vi "Dresden R2R Sputter 03.02.2018 IY24.vi"() -> ()   [LabVIEW 2009] (continued)
                      frame #2 {
                        n23216 = local read "Semi"() -> (w28558:bool)
                        n23217 = case shown="False" w28558 {
                          frame #0 {
                            n23218 = local write "RC_5"(TRUE ("RC_2")) -> ()
                            n23219 = Wait (ms)(milliseconds to wait=u32 200 ("millisecond multiple")) -> ()  [unwired: 1 out]
                          }
                          frame #1 {
                          }
                        }
                      }
                    }
                  }
                  frame #1 {
                  }
                }
              }
              frame #6 {
                # "PET COOL UP-CH2"
                n23220 = local read "Semi"() -> (w28561:bool)
                n23221 = case shown="False" w28561 {
                  frame #0 {
                    n23222 = stacked-sequence {
                      frame #0 {
                        n23223 = local read "Semi"() -> (w28562:bool)
                        n23224 = case shown="False" w28562 {
                          frame #0 {
                            n23225 = local write "Ch2_Pet_cool_down_do"(FALSE ("Ch1_pet_cool_up_do")) -> ()
                          }
                          frame #1 {
                          }
                        }
                      }
                      frame #1 {
                        n23226 = local read "Semi"() -> (w28564:bool)
                        n23227 = case shown="False" w28564 {
                          frame #0 {
                            n23228 = while {
                              i -> [w28570]
                              stop <- w28565 stop-if-true
                              n23229 = Greater?(x=w28570, y=200) -> (0:w28569:bool)
                              n23230 = case shown="True" w28569 {
                                frame #0 {
                                }
                                frame #1 {
                                n23231 = local write "Error Message"("" ("Error Message")) -> ()
                                n23232 = local write "Semi"(TRUE ("Semi")) -> ()
                                }
                              }
                              n23233 = local read "Ch2_Pet_cool_up_di"() -> (w28568:bool)
                              n23234 = case shown="False" w28568 {
                                tunnel: [FALSE TRUE] -> w28567
                                frame #0 {
                                n23235 = Wait Until Next ms Multiple(millisecond multiple=u32 200) -> ()  [unwired: 1 out]
                                n23236 = local write "Ch2_Pet_cool_up_do"(TRUE ("Ch1_pet_cool_up_do")) -> ()
                                }
                                frame #1 {
                                }
                              }
                              n23237 = local read "Semi"() -> (w28566:bool)
                              n23238 = Or(x=w28567, y=w28566) -> (x .or. y?=w28565:bool)
                            }
                          }
                          frame #1 {
                          }
                        }
                      }
                      frame #2 {
                        n23239 = local read "Semi"() -> (w28578:bool)
                        n23240 = case shown="False" w28578 {
                          frame #0 {
                            n23241 = local write "RC_6"(TRUE ("RC_2")) -> ()
                            n23242 = Wait (ms)(milliseconds to wait=u32 200 ("millisecond multiple")) -> ()  [unwired: 1 out]
                          }
                          frame #1 {
                          }
                        }
                      }
                    }
                  }
                  frame #1 {
                  }
                }
              }
              frame #7 {
                # "PET COOL UP-CH3"
                n23243 = local read "Semi"() -> (w28581:bool)
                n23244 = case shown="False" w28581 {
                  frame #0 {
                    n23245 = stacked-sequence {
                      frame #0 {
                        n23246 = local read "Semi"() -> (w28582:bool)
                        n23247 = case shown="False" w28582 {
                          frame #0 {
                            n23248 = local write "Ch3_Pet_cool_down_do"(FALSE ("Ch1_pet_cool_up_do")) -> ()
                          }
                          frame #1 {
                          }
                        }
                      }
                      frame #1 {
                        n23249 = local read "Semi"() -> (w28584:bool)
                        n23250 = case shown="False" w28584 {
                          frame #0 {
                            n23251 = while {
                              i -> [w28590]
                              stop <- w28585 stop-if-true
                              n23252 = Greater?(x=w28590, y=200) -> (0:w28589:bool)
                              n23253 = case shown="True" w28589 {
                                frame #0 {
                                }
                                frame #1 {
                                n23254 = local write "Error Message"("" ("Error Message")) -> ()
                                n23255 = local write "Semi"(TRUE ("Semi")) -> ()
                                }
                              }
                              n23256 = local read "Ch3_Pet_cool_up_di"() -> (w28588:bool)
                              n23257 = case shown="False" w28588 {
                                tunnel: [FALSE TRUE] -> w28587
                                frame #0 {
                                n23258 = Wait Until Next ms Multiple(millisecond multiple=u32 200) -> ()  [unwired: 1 out]
                                n23259 = local write "Ch3_Pet_cool_up_do"(TRUE ("Ch1_pet_cool_up_do")) -> ()
                                }
                                frame #1 {
                                }
                              }
                              n23260 = local read "Semi"() -> (w28586:bool)
                              n23261 = Or(x=w28587, y=w28586) -> (x .or. y?=w28585:bool)
                            }
                          }
                          frame #1 {
                          }
                        }
                      }
                      frame #2 {
                        n23262 = local read "Semi"() -> (w28598:bool)
                        n23263 = case shown="False" w28598 {
                          frame #0 {
                            n23264 = local write "RC_7"(TRUE ("RC_2")) -> ()
                            n23265 = Wait (ms)(milliseconds to wait=u32 200 ("millisecond multiple")) -> ()  [unwired: 1 out]
                          }
                          frame #1 {
                          }
                        }
                      }
                    }
                  }
                  frame #1 {
                  }
                }
              }
              frame #8 {
                # "PET COOL UP-CH4"
                n23266 = local read "Semi"() -> (w28601:bool)
                n23267 = case shown="False" w28601 {
                  frame #0 {
                    n23268 = stacked-sequence {
                      frame #0 {
                        n23269 = local read "Semi"() -> (w28602:bool)
                        n23270 = case shown="False" w28602 {
                          frame #0 {
                            n23271 = local write "Ch4_Pet_cool_down_do"(FALSE ("Ch1_pet_cool_up_do")) -> ()
                          }
                          frame #1 {
                          }
                        }
                      }
                      frame #1 {
                        n23272 = local read "Semi"() -> (w28604:bool)
                        n23273 = case shown="False" w28604 {
                          frame #0 {
                            n23274 = while {
                              i -> [w28610]
                              stop <- w28605 stop-if-true
                              n23275 = Greater?(x=w28610, y=200) -> (0:w28609:bool)
                              n23276 = case shown="True" w28609 {
                                frame #0 {
                                }
                                frame #1 {
                                n23277 = local write "Error Message"("" ("Error Message")) -> ()
                                n23278 = local write "Semi"(TRUE ("Semi")) -> ()
                                }
                              }
                              n23279 = local read "Ch4_Pet_cool_up_di"() -> (w28608:bool)
                              n23280 = case shown="False" w28608 {
                                tunnel: [FALSE TRUE] -> w28607
                                frame #0 {
                                n23281 = Wait Until Next ms Multiple(millisecond multiple=u32 200) -> ()  [unwired: 1 out]
                                n23282 = local write "Ch4_Pet_cool_up_do"(TRUE ("Ch1_pet_cool_up_do")) -> ()
                                }
                                frame #1 {
                                }
                              }
                              n23283 = local read "Semi"() -> (w28606:bool)
                              n23284 = Or(x=w28607, y=w28606) -> (x .or. y?=w28605:bool)
                            }
                          }
                          frame #1 {
                          }
                        }
                      }
                      frame #2 {
                        n23285 = local read "Semi"() -> (w28618:bool)
                        n23286 = case shown="False" w28618 {
                          frame #0 {
                            n23287 = local write "RC_8"(TRUE ("RC_2")) -> ()
                            n23288 = Wait (ms)(milliseconds to wait=u32 200 ("millisecond multiple")) -> ()  [unwired: 1 out]
                          }
                          frame #1 {
                          }
                        }
                      }
                    }
                  }
                  frame #1 {
                  }
                }
              }
              frame #9 {
                # "CST FIX-UP CH1"
                n23289 = local read "Semi"() -> (w28621:bool)
                n23290 = case shown="False" w28621 {
                  frame #0 {
                    n23291 = stacked-sequence {
                      frame #0 {
                        n23292 = local read "Semi"() -> (w28622:bool)
                        n23293 = case shown="False" w28622 {
                          frame #0 {
                            n23294 = while {
                              i -> [w28628]
                              stop <- w28623 stop-if-true
                              n23295 = Greater?(x=w28628, y=100) -> (0:w28627:bool)
                              n23296 = case shown="True" w28627 {
                                frame #0 {
                                }
                                frame #1 {
                                n23297 = local write "Error Message"("" ("Error Message")) -> ()
                                n23298 = local write "Semi"(TRUE ("Semi")) -> ()
                                }
                              }
                              n23299 = local read "Ch1_Cst_fix_up_di"() -> (w28626:bool)
                              n23300 = case shown="True" w28626 {
                                tunnel: [FALSE TRUE] -> w28625
                                frame #0 {
                                n23301 = Wait Until Next ms Multiple(millisecond multiple=u32 200) -> ()  [unwired: 1 out]
                                n23302 = local write "Ch1_Cst_fix_do"(FALSE ("Ch1_pet_cool_up_do")) -> ()
                                }
                                frame #1 {
                                }
                              }
                              n23303 = local read "Semi"() -> (w28624:bool)
                              n23304 = Or(x=w28625, y=w28624) -> (x .or. y?=w28623:bool)
                            }
                          }
                          frame #1 {
                          }
                        }
                      }
                      frame #1 {
                        n23305 = local read "Semi"() -> (w28636:bool)
                        n23306 = case shown="False" w28636 {
                          frame #0 {
                            n23307 = Wait (ms)(milliseconds to wait=u32 200 ("millisecond multiple")) -> ()  [unwired: 1 out]
                            n23308 = local write "RC_9"(TRUE ("RC_2")) -> ()
                          }
                          frame #1 {
                          }
                        }
                      }
                    }
                  }
                  frame #1 {
                  }
                }
              }
              frame #10 {
                # "CST FIX-UP CH2"
                n23309 = local read "Semi"() -> (w28639:bool)
                n23310 = case shown="False" w28639 {
                  frame #0 {
                    n23311 = stacked-sequence {
                      frame #0 {
                        n23312 = local read "Semi"() -> (w28640:bool)
                        n23313 = case shown="False" w28640 {
                          frame #0 {
                            n23314 = while {
                              i -> [w28646]
                              stop <- w28641 stop-if-true
                              n23315 = Greater?(x=w28646, y=100) -> (0:w28645:bool)
                              n23316 = case shown="True" w28645 {
                                frame #0 {
                                }
                                frame #1 {
                                n23317 = local write "Error Message"("" ("Error Message")) -> ()
                                n23318 = local write "Semi"(TRUE ("Semi")) -> ()
                                }
                              }
                              n23319 = local read "Ch2_Cst_fix_up_di"() -> (w28644:bool)
                              n23320 = case shown="False" w28644 {
                                tunnel: [FALSE TRUE] -> w28643
                                frame #0 {
                                n23321 = Wait Until Next ms Multiple(millisecond multiple=u32 200) -> ()  [unwired: 1 out]
                                n23322 = local write "Ch2_Cst_fix_do"(FALSE ("Ch1_pet_cool_up_do")) -> ()
                                }
                                frame #1 {
                                }
                              }
                              n23323 = local read "Semi"() -> (w28642:bool)
                              n23324 = Or(x=w28643, y=w28642) -> (x .or. y?=w28641:bool)
                            }
                          }
                          frame #1 {
                          }
                        }
                      }
                      frame #1 {
                        n23325 = local read "Semi"() -> (w28654:bool)
                        n23326 = case shown="False" w28654 {
                          frame #0 {
                            n23327 = local write "RC_10"(TRUE ("RC_2")) -> ()
                            n23328 = Wait (ms)(milliseconds to wait=u32 200 ("millisecond multiple")) -> ()  [unwired: 1 out]
                          }
                          frame #1 {
                          }
                        }
                      }
                    }
                  }
                  frame #1 {
                  }
                }
              }
              frame #11 {
                # "CST FIX-UP CH3"
                n23329 = local read "Semi"() -> (w28657:bool)
                n23330 = case shown="False" w28657 {
                  frame #0 {
                    n23331 = stacked-sequence {
                      frame #0 {
                        n23332 = local read "Semi"() -> (w28658:bool)
                        n23333 = case shown="False" w28658 {
                          frame #0 {
                            n23334 = while {
                              i -> [w28664]
                              stop <- w28659 stop-if-true
                              n23335 = Greater?(x=w28664, y=100) -> (0:w28663:bool)
                              n23336 = case shown="True" w28663 {
                                frame #0 {
                                }
                                frame #1 {
                                n23337 = local write "Error Message"("" ("Error Message")) -> ()
                                n23338 = local write "Semi"(TRUE ("Semi")) -> ()
                                }
                              }
                              n23339 = local read "Ch3_Cst_fix_up_di"() -> (w28662:bool)
                              n23340 = case shown="False" w28662 {
                                tunnel: [FALSE TRUE] -> w28661
                                frame #0 {
                                n23341 = Wait Until Next ms Multiple(millisecond multiple=u32 200) -> ()  [unwired: 1 out]
                                n23342 = local write "Ch3_Cst_fix_do"(FALSE ("Ch1_pet_cool_up_do")) -> ()
                                }
                                frame #1 {
                                }
                              }
                              n23343 = local read "Semi"() -> (w28660:bool)
                              n23344 = Or(x=w28661, y=w28660) -> (x .or. y?=w28659:bool)
                            }
                          }
                          frame #1 {
                          }
                        }
                      }
                      frame #1 {
                        n23345 = local read "Semi"() -> (w28672:bool)
                        n23346 = case shown="False" w28672 {
                          frame #0 {
                            n23347 = local write "RC_11"(TRUE ("RC_2")) -> ()
                            n23348 = Wait (ms)(milliseconds to wait=u32 200 ("millisecond multiple")) -> ()  [unwired: 1 out]
                          }
                          frame #1 {
                          }
                        }
                      }
                    }
                  }
                  frame #1 {
                  }
                }
              }
              frame #12 {
                # "CST FIX-UP CH4"
                n23349 = local read "Semi"() -> (w28675:bool)
                n23350 = case shown="False" w28675 {
                  frame #0 {
                    n23351 = stacked-sequence {
                      frame #0 {
                        n23352 = local read "Semi"() -> (w28676:bool)
                        n23353 = case shown="False" w28676 {
                          frame #0 {
                            n23354 = while {
                              i -> [w28682]
                              stop <- w28677 stop-if-true
                              n23355 = Greater?(x=w28682, y=100) -> (0:w28681:bool)
                              n23356 = case shown="True" w28681 {
                                frame #0 {
                                }
                                frame #1 {
                                n23357 = local write "Error Message"("" ("Error Message")) -> ()
                                n23358 = local write "Semi"(TRUE ("Semi")) -> ()
                                }
                              }
                              n23359 = local read "Ch4_Cst_fix_up_di"() -> (w28680:bool)
                              n23360 = case shown="False" w28680 {
                                tunnel: [FALSE TRUE] -> w28679
                                frame #0 {
                                n23361 = Wait Until Next ms Multiple(millisecond multiple=u32 200) -> ()  [unwired: 1 out]
                                n23362 = local write "Ch4_Cst_fix_do"(FALSE ("Ch1_pet_cool_up_do")) -> ()
                                }
                                frame #1 {
                                }
                              }
                              n23363 = local read "Semi"() -> (w28678:bool)
                              n23364 = Or(x=w28679, y=w28678) -> (x .or. y?=w28677:bool)
                            }
                          }
                          frame #1 {
                          }
                        }
                      }
                      frame #1 {
                        n23365 = local read "Semi"() -> (w28690:bool)
                        n23366 = case shown="False" w28690 {
                          frame #0 {
                            n23367 = Wait (ms)(milliseconds to wait=u32 200 ("millisecond multiple")) -> ()  [unwired: 1 out]
                            n23368 = local write "RC_12"(TRUE ("RC_2")) -> ()
                          }
                          frame #1 {
                          }
                        }
                      }
                      frame #2 {
                        n23369 = local read "Semi"() -> (w28693:bool)
                        n23370 = case shown="False" w28693 {
                          frame #0 {
                            n23371 = local write "Routine_check_transfer"(FALSE ("Routine_check_transfer")) -> ()
                            n23372 = Wait (ms)(milliseconds to wait=u32 200 ("millisecond multiple")) -> ()  [unwired: 1 out]
                          }
                          frame #1 {
                          }
                        }
                      }
                    }
                  }
                  frame #1 {
                  }
                }
              }
            }
          }
          frame #1 {
          }
        }
      }
    }
  }
  n23373 = while {
    stop <- FALSE stop-if-true
    n23374 = Wait Until Next ms Multiple(millisecond multiple=u32 300) -> ()  [unwired: 1 out]
    n23375 = case shown="True" "Couple" {
      frame #0 {
      }
      frame #1 {
        n23376 = stacked-sequence {
          frame #0 {
            n23377 = local read "Semi"() -> (w28744:bool)
            n23378 = case shown="False" w28744 {
              frame #0 {
                n23379 = while {
                  i -> [w28751]
                  stop <- w28746 stop-if-true
                  n23380 = Greater?(x=w28751, y=50) -> (0:w28749:bool)
                  n23381 = local read "Ch1_Cst_fix_down_di"() -> (w28745:bool)
                  n23382 = case shown="True" w28749 {
                    frame #0 {
                    }
                    frame #1 {
                      n23383 = local write "Semi"(TRUE ("Semi")) -> ()
                      n23384 = local write "Error Message"("Up/Down positions could not reach\nthe down position.\nPlease check connections." ("Error Message")) -> ()
                    }
                  }
                  n23385 = case shown="False" w28745 {
                    tunnel: [FALSE TRUE] -> w28748
                    frame #0 {
                      n23386 = Wait Until Next ms Multiple(millisecond multiple=u32 200) -> ()  [unwired: 1 out]
                      n23387 = local write "Ch1_Cst_fix_do"(TRUE ("Ch1_pet_cool_up_do")) -> ()
                    }
                    frame #1 {
                    }
                  }
                  n23388 = local read "Semi"() -> (w28747:bool)
                  n23389 = Or(x=w28748, y=w28747) -> (x .or. y?=w28746:bool)
                }
              }
              frame #1 {
              }
            }
          }
          frame #1 {
            n23390 = local read "Semi"() -> (w28758:bool)
            n23391 = case shown="False" w28758 {
              frame #0 {
                n23392 = local write "Ch1_Pet_cool_up_do"(FALSE ("Ch1_pet_cool_up_do")) -> ()
              }
              frame #1 {
              }
            }
          }
          frame #2 {
            n23393 = while {
              i -> [w28766]
              stop <- w28761 stop-if-true
              n23394 = Greater?(x=w28766, y=300) -> (0:w28764:bool)
              n23395 = case shown="True" w28764 {
                frame #0 {
                }
                frame #1 {
                  n23396 = local write "Semi"(TRUE ("Semi")) -> ()
                  n23397 = local write "Error Message"("SBS Cool Up/Down positions could not reach\nthe down position.\nPlease check connections." ("Error Message")) -> ()
                }
              }
              n23398 = local read "Ch1_Pet_cool_down_di"() -> (w28760:bool)
              n23399 = case shown="False" w28760 {
                tunnel: [FALSE TRUE] -> w28763
                frame #0 {
                  n23400 = Wait Until Next ms Multiple(millisecond multiple=u32 200) -> ()  [unwired: 1 out]
                  n23401 = local write "Ch1_Pet_cool_down_do"(TRUE ("Ch1_pet_cool_up_do")) -> ()
                }
                frame #1 {
                }
              }
              n23402 = local read "Semi"() -> (w28762:bool)
              n23403 = Or(x=w28763, y=w28762) -> (x .or. y?=w28761:bool)
            }
          }
          frame #3 {
            n23404 = local read "Semi"() -> (w28773:bool)
            n23405 = case shown="False" w28773 {
              frame #0 {
                n23406 = local write "Ch1_SRV1_PIST_Back_do"(FALSE ("Ch1_pet_cool_up_do")) -> ()
              }
              frame #1 {
              }
            }
          }
          frame #4 {
            n23407 = while {
              i -> [w28780]
              stop <- w28775 stop-if-true
              n23408 = Greater?(x=w28780, y=100) -> (0:w28779:bool)
              n23409 = case shown="True" w28779 {
                frame #0 {
                }
                frame #1 {
                  n23410 = local write "Error Message"("" ("Error Message")) -> ()
                  n23411 = local write "Semi"(TRUE ("Semi")) -> ()
                }
              }
              n23412 = local read "Ch1_SRV1_PIST For_di"() -> (w28778:bool)
              n23413 = case shown="False" w28778 {
                tunnel: [FALSE TRUE] -> w28777
                frame #0 {
                  n23414 = local write "Ch1_SRV1_PIST For_do"(TRUE ("Ch1_pet_cool_up_do")) -> ()
                  n23415 = Wait Until Next ms Multiple(millisecond multiple=u32 200) -> ()  [unwired: 1 out]
                }
                frame #1 {
                }
              }
              n23416 = local read "Semi"() -> (w28776:bool)
              n23417 = Or(x=w28777, y=w28776) -> (x .or. y?=w28775:bool)
            }
          }
        }
      }
    }
    n23418 = case shown="True" "Decouple" {
      frame #0 {
      }
      frame #1 {
        n23419 = stacked-sequence {
          frame #0 {
            n23420 = local read "Semi"() -> (w28700:bool)
            n23421 = case shown="False" w28700 {
              frame #0 {
                n23422 = while {
                  i -> [w28707]
                  stop <- w28702 stop-if-true
                  n23423 = Greater?(x=w28707, y=50) -> (0:w28705:bool)
                  n23424 = local read "Ch1_Cst_fix_up_di"() -> (w28701:bool)
                  n23425 = case shown="True" w28705 {
                    frame #0 {
                    }
                    frame #1 {
                      n23426 = local write "Semi"(TRUE ("Semi")) -> ()
                      n23427 = local write "Error Message"("Up/Down positions could not reach\nthe down position.\nPlease check connections." ("Error Message")) -> ()
                    }
                  }
                  n23428 = case shown="False" w28701 {
                    tunnel: [FALSE TRUE] -> w28704
                    frame #0 {
                      n23429 = Wait Until Next ms Multiple(millisecond multiple=u32 200) -> ()  [unwired: 1 out]
                      n23430 = local write "Ch1_Cst_fix_do"(FALSE ("Ch1_pet_cool_up_do")) -> ()
                    }
                    frame #1 {
                    }
                  }
                  n23431 = local read "Semi"() -> (w28703:bool)
                  n23432 = Or(x=w28704, y=w28703) -> (x .or. y?=w28702:bool)
                }
              }
              frame #1 {
              }
            }
          }
          frame #1 {
            n23433 = local read "Semi"() -> (w28714:bool)
            n23434 = case shown="False" w28714 {
              frame #0 {
                n23435 = local write "Ch1_Pet_cool_down_do"(FALSE ("Ch1_pet_cool_up_do")) -> ()
              }
              frame #1 {
              }
            }
          }
          frame #2 {
            n23436 = while {
              i -> [w28722]
              stop <- w28717 stop-if-true
              n23437 = Greater?(x=w28722, y=300) -> (0:w28720:bool)
              n23438 = case shown="True" w28720 {
                frame #0 {
                }
                frame #1 {
                  n23439 = local write "Semi"(TRUE ("Semi")) -> ()
                  n23440 = local write "Error Message"("SBS Cool Up/Down positions could not reach\nthe down position.\nPlease check connections." ("Error Message")) -> ()
                }
              }
              n23441 = local read "Ch1_Pet_cool_up_di"() -> (w28716:bool)
              n23442 = case shown="False" w28716 {
                tunnel: [FALSE TRUE] -> w28719
                frame #0 {
                  n23443 = Wait Until Next ms Multiple(millisecond multiple=u32 200) -> ()  [unwired: 1 out]
                  n23444 = local write "Ch1_Pet_cool_up_do"(TRUE ("Ch1_pet_cool_up_do")) -> ()
                }
                frame #1 {
                }
              }
              n23445 = local read "Semi"() -> (w28718:bool)
              n23446 = Or(x=w28719, y=w28718) -> (x .or. y?=w28717:bool)
            }
          }
          frame #3 {
            n23447 = local read "Semi"() -> (w28729:bool)
            n23448 = case shown="False" w28729 {
              frame #0 {
                n23449 = local write "Ch1_SRV1_PIST For_do"(FALSE ("Ch1_pet_cool_up_do")) -> ()
              }
              frame #1 {
              }
            }
          }
          frame #4 {
            n23450 = while {
              i -> [w28736]
              stop <- w28731 stop-if-true
              n23451 = Greater?(x=w28736, y=100) -> (0:w28735:bool)
              n23452 = case shown="True" w28735 {
                frame #0 {
                }
                frame #1 {
                  n23453 = local write "Error Message"("" ("Error Message")) -> ()
                  n23454 = local write "Semi"(TRUE ("Semi")) -> ()
                }
              }
              n23455 = local read "Ch1_SRV1_PIST_Back_di"() -> (w28734:bool)
              n23456 = case shown="False" w28734 {
                tunnel: [FALSE TRUE] -> w28733
                frame #0 {
                  n23457 = local write "Ch1_SRV1_PIST_Back_do"(TRUE ("Ch1_pet_cool_up_do")) -> ()
                  n23458 = Wait Until Next ms Multiple(millisecond multiple=u32 200) -> ()  [unwired: 1 out]
                }
                frame #1 {
                }
              }
              n23459 = local read "Semi"() -> (w28732:bool)
              n23460 = Or(x=w28733, y=w28732) -> (x .or. y?=w28731:bool)
            }
          }
        }
      }
    }
  }
  n23461 = VISA Close(VISA resource name=w789, error in (no error)=w788) -> ()  [unwired: 1 out]
  n23462 = while {
    stop <- i16? 0 stop-if-true
    n23463 = Wait (ms)(milliseconds to wait=i32? 300) -> ()  [unwired: 1 out]
    n23464 = stacked-sequence {
      frame #0 {
        n23465 = case shown="True" "Clean_Pumping_ch1" {
          frame #0 {
          }
          frame #1 {
            w28830 = i16? 0
            n23466 = local write "Clean_Pumping_ch1"(w28830) -> ()
            "Ch1_PV2" <- w28830
            "Ch1_PV6" <- w28830
            "Ch1_PV7" <- w28830
            "Ch1_PV8" <- w28830
            "Ch1_PV9" <- w28830
            "Ch1_PV15" <- w28830
            "Ch1_PV10" <- w28830
            "Ch1_PV16" <- w28830
            "Ch1_PV13" <- w28830
            "Ch1_PA15" <- w28830
            "Ch1_PA9" <- w28830
            "Ch1_PA10" <- w28830
            "Ch1_PA17" <- w28830
            "Ch1_PA2" <- w28830
            "Ch1_PA6" <- w28830
            "Ch1_PA7" <- w28830
            "Ch1_PA8" <- w28830
            "Ch1_PA14" <- w28830
            "Ch1_PA19" <- w28830
            "Ch1_PA20" <- w28830
            "Ch1_PA24" <- w28830
            "Ch1_PA25" <- w28830
            "Ch1_PA16" <- w28830
            "Ch1_PA18" <- w28830
            "Ch1_PA22" <- w28830
            "Ch1_PV11" <- w28830
            "Ch1_PV14" <- w28830
            "Ch1_PV19" <- w28830
            "Ch1_PV20" <- w28830
            "Ch1_PV23" <- w28830
            "Ch1_PV22" <- w28830
            "Ch1_PV4" <- w28830
            "Ch1_PV18" <- w28830
            "Ch1_PA4" <- w28830
            "Ch1_PA11" <- w28830
            "Ch1_PA13" <- w28830
            "Ch1_PA21" <- w28830
            "Ch1_PV12" <- w28830
            "Ch1_PV17" <- w28830
            "Ch1_PA26" <- w28830
            "Ch1_PA27" <- w28830
            "Ch1_PA28" <- w28830
            "Ch1_PA30" <- w28830
            "Ch1_PA29" <- w28830
            "Ch1_PA12" <- w28830
            "Ch1_PA23" <- w28830
            "Ch1_PA31" <- w28830
            "Ch1_PV3" <- w28830
            "Ch1_PA3" <- w28830
            "Ch1_PV1" <- w28830
            "Ch1_PA1" <- w28830
            "Ch1_PA5" <- w28830
            "Ch1_PV5" <- w28830
            "Ch1_PA33" <- w28830
            "Ch1_PA34" <- w28830
            "Ch1_PA32" <- w28830
            "Ch1_PV21" <- w28830
          }
        }
        n23467 = case shown="True" "Clean_shutdown_ch1" {
          frame #0 {
          }
          frame #1 {
            w28831 = i16? 0
            n23468 = local write "Clean_shutdown_ch1"(w28831) -> ()
            "Ch1_Sd0" <- w28831
            "Ch1_Sd1" <- w28831
            "Ch1_Sd3" <- w28831
            "Ch1_Sd8" <- w28831
            "Ch1_Sd6" <- w28831
            "Ch1_Sd5" <- w28831
            "Ch1_Sd14" <- w28831
            "Ch1_Sd7" <- w28831
            "Ch1_Sd10" <- w28831
            "Ch1_Sd12" <- w28831
            "Ch1_Sd11" <- w28831
            "Ch1_Sd19" <- w28831
            "Ch1_Sd4" <- w28831
            "Ch1_Sd17" <- w28831
            "Ch1_Sd2" <- w28831
            "Ch1_Sd16" <- w28831
            "Ch1_Sd18" <- w28831
            "Ch1_Sd13" <- w28831
            "Ch1_Sd15" <- w28831
            "Ch1_Sd9" <- w28831
          }
        }
      }
    }
    n23469 = stacked-sequence {
      frame #0 {
        n23470 = case shown="True" "Clean_Pumping_ch2" {
          frame #0 {
          }
          frame #1 {
            w28827 = i16? 0
            n23471 = local write "Clean_Pumping_ch2"(w28827) -> ()
            "Ch2_PA0" <- w28827
            "Ch2_PA1" <- w28827
            "Ch2_PA2" <- w28827
            "Ch2_PA3" <- w28827
            "Ch2_PA4" <- w28827
            "Ch2_PA5" <- w28827
            "Ch2_PA6" <- w28827
            "Ch2_PA7" <- w28827
            "Ch2_PA8" <- w28827
            "Ch2_PA9" <- w28827
            "Ch2_PA10" <- w28827
            "Ch2_PA11" <- w28827
            "Ch2_PA12" <- w28827
            "Ch2_PA13" <- w28827
            "Ch2_PA18" <- w28827
            "Ch2_PA14" <- w28827
            "Ch2_PA15" <- w28827
            "Ch2_PA17" <- w28827
            "Ch2_PA16" <- w28827
            "Ch2_PA19" <- w28827
            "Ch2_PA20" <- w28827
            "Ch2_PA21" <- w28827
            "Ch2_PA22" <- w28827
            "Ch2_PA23" <- w28827
            "Ch2_PA24" <- w28827
            "Ch2_PA25" <- w28827
            "Ch2_PA26" <- w28827
            "Ch2_PA27" <- w28827
            "Ch2_PA28" <- w28827
            "Ch2_PA29" <- w28827
            "Ch2_PA30" <- w28827
            "Ch2_PA31" <- w28827
            "Ch2_PA32" <- w28827
            "Ch2_PA35" <- w28827
            "Ch2_PV0" <- w28827
            "Ch2_PV1" <- w28827
            "Ch2_PV7" <- w28827
            "Ch2_PV2" <- w28827
            "Ch2_PV3" <- w28827
            "Ch2_PV4" <- w28827
            "Ch2_PV5" <- w28827
            "Ch2_PV6" <- w28827
            "Ch2_PV8" <- w28827
            "Ch2_PV9" <- w28827
            "Ch2_PV10" <- w28827
            "Ch2_PV11" <- w28827
            "Ch2_PV12" <- w28827
            "Ch2_PV13" <- w28827
            "Ch2_PV14" <- w28827
            "Ch2_PV15" <- w28827
            "Ch2_PV16" <- w28827
            "Ch2_PV17" <- w28827
            "Ch2_PV18" <- w28827
            "Ch2_PV19" <- w28827
            "Ch2_PV20" <- w28827
            "Ch2_PV24" <- w28827
            "Ch2_PV21" <- w28827
            "Ch2_PV25" <- w28827
            "Ch2_PA36" <- w28827
            "Ch2_PA33" <- w28827
            "Ch2_PA34" <- w28827
            "Ch2_PV22" <- w28827
            "Ch2_PV23" <- w28827
          }
        }
        n23472 = case shown="True" "Clean_shutdown_ch2" {
          frame #0 {
          }
          frame #1 {
            w28826 = i16? 0
            n23473 = local write "Clean_shutdown_ch2"(w28826) -> ()
            "Ch2_Sd1" <- w28826
            "Ch2_Sd3" <- w28826
            "Ch2_Sd2" <- w28826
            "Ch2_Sd4" <- w28826
            "Ch2_Sd5" <- w28826
            "Ch2_Sd7" <- w28826
            "Ch2_Sd6" <- w28826
            "Ch2_Sd8" <- w28826
            "Ch2_Sd9" <- w28826
            "Ch2_Sd10" <- w28826
            "Ch2_Sd11" <- w28826
            "Ch2_Sd12" <- w28826
            "Ch2_Sd13" <- w28826
            "Ch2_Sd14" <- w28826
            "Ch2_Sd17" <- w28826
            "Ch2_Sd18" <- w28826
            "Ch2_Sd19" <- w28826
            "Ch2_Sd20" <- w28826
            "Ch2_Sd21" <- w28826
            "Ch2_Sd22" <- w28826
            "Ch2_Sd15" <- w28826
            "Ch2_Sd16" <- w28826
          }
        }
      }
    }
    n23474 = stacked-sequence {
      frame #0 {
        n23475 = case shown="True" "Clean_Pumping_ch3" {
          frame #0 {
          }
          frame #1 {
            w28823 = i16? 0
            n23476 = local write "Clean_Pumping_ch3"(w28823) -> ()
            "Ch3_PA0" <- w28823
            "Ch3_PA1" <- w28823
            "Ch3_PA2" <- w28823
            "Ch3_PA3" <- w28823
            "Ch3_PA4" <- w28823
            "Ch3_PA5" <- w28823
            "Ch3_PA6" <- w28823
            "Ch3_PA7" <- w28823
            "Ch3_PA8" <- w28823
            "Ch3_PA9" <- w28823
            "Ch3_PA10" <- w28823
            "Ch3_PA11" <- w28823
            "Ch3_PA12" <- w28823
            "Ch3_PA13" <- w28823
            "Ch3_PA14" <- w28823
            "Ch3_PA15" <- w28823
            "Ch3_PA17" <- w28823
            "Ch3_PA18" <- w28823
            "Ch3_PA16" <- w28823
            "Ch3_PA19" <- w28823
            "Ch3_PA20" <- w28823
            "Ch3_PA22" <- w28823
            "Ch3_PA23" <- w28823
            "Ch3_PA24" <- w28823
            "Ch3_PA21" <- w28823
            "Ch3_PA26" <- w28823
            "Ch3_PA25" <- w28823
            "Ch3_PA27" <- w28823
            "Ch3_PA28" <- w28823
            "Ch3_PA29" <- w28823
            "Ch3_PA30" <- w28823
            "Ch3_PA31" <- w28823
            "Ch3_PA32" <- w28823
            "Ch3_PA35" <- w28823
            "Ch3_PA36" <- w28823
            "Ch3_PV0" <- w28823
            "Ch3_PV1" <- w28823
            "Ch3_PV2" <- w28823
            "Ch3_PV3" <- w28823
            "Ch3_PV4" <- w28823
            "Ch3_PV5" <- w28823
            "Ch3_PV6" <- w28823
            "Ch3_PV7" <- w28823
            "Ch3_PV8" <- w28823
            "Ch3_PV9" <- w28823
            "Ch3_PV10" <- w28823
            "Ch3_PV11" <- w28823
            "Ch3_PV12" <- w28823
            "Ch3_PV13" <- w28823
            "Ch3_PV14" <- w28823
            "Ch3_PV15" <- w28823
            "Ch3_PV16" <- w28823
            "Ch3_PV17" <- w28823
            "Ch3_PV18" <- w28823
            "Ch3_PV19" <- w28823
            "Ch3_PV20" <- w28823
            "Ch3_PV21" <- w28823
            "Ch3_PV24" <- w28823
            "Ch3_PV25" <- w28823
            "Ch3_PA33" <- w28823
            "Ch3_PA34" <- w28823
            "Ch3_PV22" <- w28823
            "Ch3_PV23" <- w28823
          }
        }
        n23477 = case shown="True" "Clean_shutdown_ch3" {
          frame #0 {
          }
          frame #1 {
            w28822 = i16? 0 ("Ch3_Sd0")
            n23478 = local write "Clean_shutdown_ch3"(w28822) -> ()
            "Ch3_Sd1" <- w28822
            "Ch3_Sd2" <- w28822
            "Ch3_Sd3" <- w28822
            "Ch3_Sd4" <- w28822
            "Ch3_Sd5" <- w28822
            "Ch3_Sd6" <- w28822
            "Ch3_Sd7" <- w28822
            "Ch3_Sd8" <- w28822
            "Ch3_Sd9" <- w28822
            "Ch3_Sd10" <- w28822
            "Ch3_Sd11" <- w28822
            "Ch3_Sd12" <- w28822
            "Ch3_Sd13" <- w28822
            "Ch3_Sd14" <- w28822
            "Ch3_Sd15" <- w28822
            "Ch3_Sd16" <- w28822
            "Ch3_Sd19" <- w28822
            "Ch3_Sd20" <- w28822
            "Ch3_Sd21" <- w28822
            "Ch3_Sd22" <- w28822
            "Ch3_Sd17" <- w28822
            "Ch3_Sd18" <- w28822
          }
        }
      }
    }
    n23479 = stacked-sequence {
      frame #0 {
        n23480 = case shown="True" "Clean_Pumping_ch4" {
          frame #0 {
          }
          frame #1 {
            w28819 = i16? 0
            n23481 = local write "Clean_Pumping_ch4"(w28819) -> ()
            "Ch4_PA0" <- w28819
            "Ch4_PA1" <- w28819
            "Ch4_PA2" <- w28819
            "Ch4_PA3" <- w28819
            "Ch4_PA4" <- w28819
            "Ch4_PA5" <- w28819
            "Ch4_PA6" <- w28819
            "Ch4_PA7" <- w28819
            "Ch4_PA8" <- w28819
            "Ch4_PA9" <- w28819
            "Ch4_PA10" <- w28819
            "Ch4_PA11" <- w28819
            "Ch4_PA12" <- w28819
            "Ch4_PA13" <- w28819
            "Ch4_PA14" <- w28819
            "Ch4_PA16" <- w28819
            "Ch4_PA15" <- w28819
            "Ch4_PA17" <- w28819
            "Ch4_PA18" <- w28819
            "Ch4_PA19" <- w28819
            "Ch4_PA20" <- w28819
            "Ch4_PA21" <- w28819
            "Ch4_PA22" <- w28819
            "Ch4_PA25" <- w28819
            "Ch4_PA26" <- w28819
            "Ch4_PA28" <- w28819
            "Ch4_PA27" <- w28819
            "Ch4_PA29" <- w28819
            "Ch4_PA30" <- w28819
            "Ch4_PA31" <- w28819
            "Ch4_PA32" <- w28819
            "Ch4_PA34" <- w28819
            "Ch4_PA35" <- w28819
            "Ch4_PV0" <- w28819
            "Ch4_PV1" <- w28819
            "Ch4_PV2" <- w28819
            "Ch4_PV3" <- w28819
            "Ch4_PV4" <- w28819
            "Ch4_PV5" <- w28819
            "Ch4_PV6" <- w28819
            "Ch4_PV7" <- w28819
            "Ch4_PV8" <- w28819
            "Ch4_PV9" <- w28819
            "Ch4_PV10" <- w28819
            "Ch4_PV11" <- w28819
            "Ch4_PV12" <- w28819
            "Ch4_PV13" <- w28819
            "Ch4_PV14" <- w28819
            "Ch4_PV15" <- w28819
            "Ch4_PV16" <- w28819
            "Ch4_PV17" <- w28819
            "Ch4_PV18" <- w28819
            "Ch4_PV19" <- w28819
            "Ch4_PV21" <- w28819
            "Ch4_PV22" <- w28819
            "Ch4_PA33" <- w28819
            "Ch4_PV20" <- w28819
          }
        }
        n23482 = case shown="True" "Clean_shutdown_ch4" {
          frame #0 {
          }
          frame #1 {
            w28818 = i16? 0
            n23483 = local write "Clean_shutdown_ch4"(w28818) -> ()
            "Ch4_Sd1" <- w28818
            "Ch4_Sd2" <- w28818
            "Ch4_Sd3" <- w28818
            "Ch4_Sd4" <- w28818
            "Ch4_Sd5" <- w28818
            "Ch4_Sd6" <- w28818
            "Ch4_Sd7" <- w28818
            "Ch4_Sd8" <- w28818
            "Ch4_Sd 9" <- w28818
            "Ch4_Sd10" <- w28818
            "Ch4_Sd11" <- w28818
            "Ch4_Sd12" <- w28818
            "Ch4_Sd14" <- w28818
            "Ch4_Sd13" <- w28818
            "Ch4_Sd15" <- w28818
            "Ch4_Sd17" <- w28818
            "Ch4_Sd18" <- w28818
            "Ch4_Sd19" <- w28818
            "Ch4_Sd20" <- w28818
            "Ch4_Sd16" <- w28818
          }
        }
      }
    }
    n23484 = case shown="True" "Clean_trnsfr_1_2" {
      frame #0 {
      }
      frame #1 {
        w28815 = i16? 0
        n23485 = local write "Clean_trnsfr_1_2"(w28815) -> ()
        "CH1_2_trns_1" <- w28815
        "CH1_2_trns_0" <- w28815
        "CH1_2trns_10" <- w28815
        "CH1_2trns_14" <- w28815
        "CH1_2trns_16" <- w28815
        "CH1_2trns_18" <- w28815
        "CH1_2trns_9" <- w28815
        "CH1_2trns_4" <- w28815
        "CH1_2trns_13" <- w28815
        "CH1_2trns_2" <- w28815
        "CH1_2trns_15" <- w28815
        "CH1_2trns_17" <- w28815
        "CH1_2trns_3" <- w28815
        "CH1_2trns_5" <- w28815